vi "Dresden R2R Sputter 03.02.2018 IY24.vi"() -> ()   [LabVIEW 2009] (continued)
                n995 = local write "Casette_mechanism_1"(T/1 ("Casette_mechanism_4")) -> ()
                n996 = local write "Casette_mechanism_4"(i16? 0 ("Casette_mechanism_4")) -> ()
                n997 = local write "Casette_mechanism_3"(i16? 0 ("Casette_mechanism_3")) -> ()
                n998 = local write "Casette_mechanism_2"(i16? 0 ("Casette_mechanism_2")) -> ()
                "Ch1_tab_led" <- T/1 ("Ch1_tab_led")
                "Ch1_pump_tab_led" <- T/1 ("Ch1_pump_tab_led")
              }
              frame #2 {
                n999 = local write "ch_present_position"(dbl? 2.0 ("ch_present_position")) -> ()
                n1000 = local write "Casette_mechanism_2"(T/1 ("Casette_mechanism_2")) -> ()
                n1001 = local write "Casette_mechanism_1"(i16? 0 ("Casette_mechanism_4")) -> ()
                n1002 = local write "Casette_mechanism_4"(i16? 0 ("Casette_mechanism_4")) -> ()
                n1003 = local write "Casette_mechanism_3"(i16? 0 ("Casette_mechanism_3")) -> ()
                "Ch2_tab_led" <- T/1 ("Ch2_tab_led")
                "Ch2_pump_tab_led" <- T/1 ("Ch2_pump_tab_led")
              }
              frame #3 {
                n1004 = local write "ch_present_position"(dbl? 3.0 ("ch_present_position")) -> ()
                n1005 = local write "Casette_mechanism_3"(T/1 ("Casette_mechanism_3")) -> ()
                n1006 = local write "Casette_mechanism_2"(i16? 0 ("Casette_mechanism_2")) -> ()
                n1007 = local write "Casette_mechanism_1"(i16? 0 ("Casette_mechanism_4")) -> ()
                n1008 = local write "Casette_mechanism_4"(i16? 0 ("Casette_mechanism_4")) -> ()
                "Ch3_tab_led" <- T/1 ("Ch3_tab_led")
                "Ch3_pump_tab_led" <- T/1 ("Ch3_pump_tab_led")
              }
              frame #4 {
                n1009 = local write "ch_present_position"(dbl? 4.0 ("ch_present_position")) -> ()
                n1010 = local write "Casette_mechanism_4"(T/1 ("Casette_mechanism_4")) -> ()
                n1011 = local write "Casette_mechanism_3"(i16? 0 ("Casette_mechanism_3")) -> ()
                n1012 = local write "Casette_mechanism_2"(i16? 0 ("Casette_mechanism_2")) -> ()
                n1013 = local write "Casette_mechanism_1"(i16? 0 ("Casette_mechanism_4")) -> ()
                "Ch4_tab_led" <- T/1 ("Ch4_tab_led")
                "Ch4_pump_tab_led" <- T/1 ("Ch4_pump_tab_led")
              }
            }
            n1014 = Mantissa & Exponent(0:w1015) -> (2:w1013)  [unwired: 1 out]
            n1015 = case shown="1" w1013 {
              tunnel: [w1048 "Left" ("Casette_direction") "Right" ("Casette_direction")] -> w1012
              frame #0 {
                n1016 = local read "Casette_direction"() -> (w1048)
              }
              frame #1 {
              }
              frame #2 {
              }
            }
            "Casette_direction" <- w1012
          }
        }
      }
    }
  }
  n1017 = Build Path(base path="Gui_path", name or relative path="bv4 on.jpg") -> (appended path=w600:path)
  n1018 = Build Path(base path="Gui_path", name or relative path="bv4 fail.jpg") -> (appended path=w597:path)
  n1019 = Build Path(base path="Gui_path", name or relative path="gv on.jpg") -> (appended path=w605:path)
  n1020 = Build Path(base path="Gui_path", name or relative path="gv fail.jpg") -> (appended path=w608:path)
  n1021 = Build Path(base path="Gui_path", name or relative path="bv1 on.jpg") -> (appended path=w648:path)
  n1022 = Build Path(base path="Gui_path", name or relative path="vbv on.jpg") -> (appended path=w715:path)
  n1023 = Build Path(base path="Gui_path", name or relative path="bv1 fail.jpg") -> (appended path=w645:path)
  n1024 = Build Path(base path="Gui_path", name or relative path="mp on.jpg") -> (appended path=w728:path)
  n1025 = Build Path(base path="Gui_path", name or relative path="vbv fail.jpg") -> (appended path=w718:path)
  n1026 = Build Path(base path="Gui_path", name or relative path="mp fail.jpg") -> (appended path=w725:path)
  n1027 = Build Path(base path="Gui_path", name or relative path="pg on.jpg") -> (appended path=w712:path)
  n1028 = Build Path(base path="Gui_path", name or relative path="pg fail.jpg") -> (appended path=w709:path)
  n1029 = Build Path(base path="Gui_path", name or relative path="atm2 on.jpg") -> (appended path=w699:path)
  n1030 = Build Path(base path="Gui_path", name or relative path="atm2 fail.jpg") -> (appended path=w702:path)
  n1031 = Build Path(base path="Gui_path", name or relative path="bv1 on.jpg") -> (appended path=w696:path)
  n1032 = Build Path(base path="Gui_path", name or relative path="bv1 fail.jpg") -> (appended path=w693:path)
  n1033 = Build Path(base path="Gui_path", name or relative path="bv3 on.jpg") -> (appended path=w621:path)
  n1034 = Build Path(base path="Gui_path", name or relative path="vbv on.jpg") -> (appended path=w683:path)
  n1035 = Build Path(base path="Gui_path", name or relative path="bv3 fail.jpg") -> (appended path=w624:path)
  n1036 = Build Path(base path="Gui_path", name or relative path="vbv fail.jpg") -> (appended path=w686:path)
  n1037 = Build Path(base path="Gui_path", name or relative path="tp on.jpg") -> (appended path=w680:path)
  n1038 = Build Path(base path="Gui_path", name or relative path="tp fail.jpg") -> (appended path=w677:path)
  n1039 = Build Path(base path="Gui_path", name or relative path="tp gv on.jpg") -> (appended path=w667:path)
  n1040 = Build Path(base path="Gui_path", name or relative path="pg2 on.jpg") -> (appended path=w664:path)
  n1041 = Build Path(base path="Gui_path", name or relative path="tp gv fail.jpg") -> (appended path=w670:path)
  n1042 = Build Path(base path="Gui_path", name or relative path="tp gv middle.jpg") -> (appended path=w49:path)
  n1043 = Build Path(base path="Gui_path", name or relative path="pg2 fail.jpg") -> (appended path=w661:path)
  n1044 = Build Path(base path="Gui_path", name or relative path="bv2 on.jpg") -> (appended path=w618:path)
  n1045 = Build Path(base path="Gui_path", name or relative path="bv2 fail.jpg") -> (appended path=w615:path)
  n1046 = Build Path(base path="Gui_path", name or relative path="brt on.jpg") -> (appended path=w635:path)
  n1047 = Build Path(base path="Gui_path", name or relative path="brt fail.jpg") -> (appended path=w638:path)
  n1048 = Build Path(base path="Gui_path", name or relative path="atm3 on.jpg") -> (appended path=w632:path)
  n1049 = Build Path(base path="Gui_path", name or relative path="atm3 fail.jpg") -> (appended path=w629:path)
  n1050 = Build Path(base path="Gui_path", name or relative path="cc on.jpg") -> (appended path=w651:path)
  n1051 = Build Path(base path="Gui_path", name or relative path="cc fail.jpg") -> (appended path=w654:path)
  n1052 = Build Path(base path="Gui_path", name or relative path="bv5 on.jpg") -> (appended path=w591:path)
  n1053 = Build Path(base path="Gui_path", name or relative path="bv5 fail.jpg") -> (appended path=w594:path)
  n1054 = Build Path(base path="Gui_path", name or relative path="casette mechanism.jpg") -> (appended path=w42:path)
  n1055 = call <vilib>:"Read JPEG File.vi"("path to JPEG file"=w600) -> ("image data"=w601:T34)  [unwired: 8 in, 2 out]
  n1056 = call <vilib>:"Read JPEG File.vi"("path to JPEG file"=w597) -> ("image data"=w596:T34)  [unwired: 8 in, 2 out]
  n1057 = call <vilib>:"Read JPEG File.vi"("path to JPEG file"="Background_path") -> ("image data"=w732:T34)  [unwired: 8 in, 2 out]
  n1058 = call <vilib>:"Read JPEG File.vi"("path to JPEG file"=w605) -> ("image data"=w604:T34)  [unwired: 8 in, 2 out]
  n1059 = call <vilib>:"Read JPEG File.vi"("path to JPEG file"=w608) -> ("image data"=w609:T34)  [unwired: 8 in, 2 out]
  n1060 = call <vilib>:"Read JPEG File.vi"("path to JPEG file"=w648) -> ("image data"=w649:T34)  [unwired: 8 in, 2 out]
  n1061 = call <vilib>:"Read JPEG File.vi"("path to JPEG file"=w715) -> ("image data"=w714:T34)  [unwired: 8 in, 2 out]
  n1062 = call <vilib>:"Read JPEG File.vi"("path to JPEG file"=w645) -> ("image data"=w644:T34)  [unwired: 8 in, 2 out]
  n1063 = call <vilib>:"Read JPEG File.vi"("path to JPEG file"=w728) -> ("image data"=w729:T34)  [unwired: 8 in, 2 out]
  n1064 = call <vilib>:"Read JPEG File.vi"("path to JPEG file"=w718) -> ("image data"=w719:T34)  [unwired: 8 in, 2 out]
  n1065 = call <vilib>:"Read JPEG File.vi"("path to JPEG file"=w725) -> ("image data"=w724:T34)  [unwired: 8 in, 2 out]
  n1066 = call <vilib>:"Read JPEG File.vi"("path to JPEG file"=w712) -> ("image data"=w713:T34)  [unwired: 8 in, 2 out]
  n1067 = call <vilib>:"Read JPEG File.vi"("path to JPEG file"=w709) -> ("image data"=w708:T34)  [unwired: 8 in, 2 out]
  n1068 = call <vilib>:"Read JPEG File.vi"("path to JPEG file"=w699) -> ("image data"=w698:T34)  [unwired: 8 in, 2 out]
  n1069 = call <vilib>:"Read JPEG File.vi"("path to JPEG file"=w702) -> ("image data"=w703:T34)  [unwired: 8 in, 2 out]
  n1070 = call <vilib>:"Read JPEG File.vi"("path to JPEG file"=w696) -> ("image data"=w697:T34)  [unwired: 8 in, 2 out]
  n1071 = call <vilib>:"Read JPEG File.vi"("path to JPEG file"=w693) -> ("image data"=w692:T34)  [unwired: 8 in, 2 out]
  n1072 = call <vilib>:"Read JPEG File.vi"("path to JPEG file"=w621) -> ("image data"=w620:T34)  [unwired: 8 in, 2 out]
  n1073 = call <vilib>:"Read JPEG File.vi"("path to JPEG file"=w683) -> ("image data"=w682:T34)  [unwired: 8 in, 2 out]
  n1074 = call <vilib>:"Read JPEG File.vi"("path to JPEG file"=w624) -> ("image data"=w625:T34)  [unwired: 8 in, 2 out]
  n1075 = call <vilib>:"Read JPEG File.vi"("path to JPEG file"=w686) -> ("image data"=w687:T34)  [unwired: 8 in, 2 out]
  n1076 = call <vilib>:"Read JPEG File.vi"("path to JPEG file"=w680) -> ("image data"=w681:T34)  [unwired: 8 in, 2 out]
  n1077 = call <vilib>:"Read JPEG File.vi"("path to JPEG file"=w677) -> ("image data"=w676:T34)  [unwired: 8 in, 2 out]
  n1078 = call <vilib>:"Read JPEG File.vi"("path to JPEG file"=w667) -> ("image data"=w666:T34)  [unwired: 8 in, 2 out]
  n1079 = call <vilib>:"Read JPEG File.vi"("path to JPEG file"=w664) -> ("image data"=w665:T34)  [unwired: 8 in, 2 out]
  n1080 = call <vilib>:"Read JPEG File.vi"("path to JPEG file"=w670) -> ("image data"=w671:T34)  [unwired: 8 in, 2 out]
  n1081 = call <vilib>:"Read JPEG File.vi"("path to JPEG file"=w49) -> ("image data"=w48:T34)  [unwired: 8 in, 2 out]
  n1082 = call <vilib>:"Read JPEG File.vi"("path to JPEG file"=w661) -> ("image data"=w660:T34)  [unwired: 8 in, 2 out]
  n1083 = call <vilib>:"Read JPEG File.vi"("path to JPEG file"=w618) -> ("image data"=w619:T34)  [unwired: 8 in, 2 out]
  n1084 = call <vilib>:"Read JPEG File.vi"("path to JPEG file"=w615) -> ("image data"=w614:T34)  [unwired: 8 in, 2 out]
  n1085 = call <vilib>:"Read JPEG File.vi"("path to JPEG file"=w635) -> ("image data"=w634:T34)  [unwired: 8 in, 2 out]
  n1086 = call <vilib>:"Read JPEG File.vi"("path to JPEG file"=w638) -> ("image data"=w639:T34)  [unwired: 8 in, 2 out]
  n1087 = call <vilib>:"Read JPEG File.vi"("path to JPEG file"=w632) -> ("image data"=w633:T34)  [unwired: 8 in, 2 out]
  n1088 = call <vilib>:"Read JPEG File.vi"("path to JPEG file"=w629) -> ("image data"=w628:T34)  [unwired: 8 in, 2 out]
  n1089 = call <vilib>:"Read JPEG File.vi"("path to JPEG file"=w651) -> ("image data"=w650:T34)  [unwired: 8 in, 2 out]
  n1090 = call <vilib>:"Read JPEG File.vi"("path to JPEG file"=w654) -> ("image data"=w655:T34)  [unwired: 8 in, 2 out]
  n1091 = call <vilib>:"Read JPEG File.vi"("path to JPEG file"=w591) -> ("image data"=w590:T34)  [unwired: 8 in, 2 out]
  n1092 = call <vilib>:"Read JPEG File.vi"("path to JPEG file"=w594) -> ("image data"=w595:T34)  [unwired: 8 in, 2 out]
  n1093 = call <vilib>:"Read JPEG File.vi"("path to JPEG file"=w42) -> ("image data"=w45:T34)  [unwired: 8 in, 2 out]
  n1094 = call <vilib>:"Unflatten Pixmap.vi"("image data"=w601) -> ("24-bit pixmap"=w589:u32[][])  [unwired: 4 in, 6 out]
  n1095 = call <vilib>:"Unflatten Pixmap.vi"("image data"=w596) -> ("24-bit pixmap"=w588:u32[][])  [unwired: 4 in, 6 out]
  n1096 = call <vilib>:"Unflatten Pixmap.vi"("image data"=w732) -> ("24-bit pixmap"=w730:u32[][])  [unwired: 4 in, 6 out]
  n1097 = call <vilib>:"Unflatten Pixmap.vi"("image data"=w604) -> ("24-bit pixmap"=w603:u32[][])  [unwired: 4 in, 6 out]
  n1098 = call <vilib>:"Unflatten Pixmap.vi"("image data"=w609) -> ("24-bit pixmap"=w602:u32[][])  [unwired: 4 in, 6 out]
  n1099 = call <vilib>:"Unflatten Pixmap.vi"("image data"=w649) -> ("24-bit pixmap"=w643:u32[][])  [unwired: 4 in, 6 out]
  n1100 = call <vilib>:"Unflatten Pixmap.vi"("image data"=w714) -> ("24-bit pixmap"=w720:u32[][])  [unwired: 4 in, 6 out]
  n1101 = call <vilib>:"Unflatten Pixmap.vi"("image data"=w644) -> ("24-bit pixmap"=w642:u32[][])  [unwired: 4 in, 6 out]
  n1102 = call <vilib>:"Unflatten Pixmap.vi"("image data"=w729) -> ("24-bit pixmap"=w723:u32[][])  [unwired: 4 in, 6 out]
  n1103 = call <vilib>:"Unflatten Pixmap.vi"("image data"=w719) -> ("24-bit pixmap"=w721:u32[][])  [unwired: 4 in, 6 out]
  n1104 = call <vilib>:"Unflatten Pixmap.vi"("image data"=w724) -> ("24-bit pixmap"=w722:u32[][])  [unwired: 4 in, 6 out]
  n1105 = call <vilib>:"Unflatten Pixmap.vi"("image data"=w713) -> ("24-bit pixmap"=w707:u32[][])  [unwired: 4 in, 6 out]
  n1106 = call <vilib>:"Unflatten Pixmap.vi"("image data"=w708) -> ("24-bit pixmap"=w706:u32[][])  [unwired: 4 in, 6 out]
  n1107 = call <vilib>:"Unflatten Pixmap.vi"("image data"=w698) -> ("24-bit pixmap"=w704:u32[][])  [unwired: 4 in, 6 out]
  n1108 = call <vilib>:"Unflatten Pixmap.vi"("image data"=w703) -> ("24-bit pixmap"=w705:u32[][])  [unwired: 4 in, 6 out]
  n1109 = call <vilib>:"Unflatten Pixmap.vi"("image data"=w697) -> ("24-bit pixmap"=w691:u32[][])  [unwired: 4 in, 6 out]
  n1110 = call <vilib>:"Unflatten Pixmap.vi"("image data"=w692) -> ("24-bit pixmap"=w690:u32[][])  [unwired: 4 in, 6 out]
  n1111 = call <vilib>:"Unflatten Pixmap.vi"("image data"=w682) -> ("24-bit pixmap"=w688:u32[][])  [unwired: 4 in, 6 out]
  n1112 = call <vilib>:"Unflatten Pixmap.vi"("image data"=w687) -> ("24-bit pixmap"=w689:u32[][])  [unwired: 4 in, 6 out]
  n1113 = call <vilib>:"Unflatten Pixmap.vi"("image data"=w681) -> ("24-bit pixmap"=w675:u32[][])  [unwired: 4 in, 6 out]
  n1114 = call <vilib>:"Unflatten Pixmap.vi"("image data"=w620) -> ("24-bit pixmap"=w613:u32[][])  [unwired: 4 in, 6 out]
  n1115 = call <vilib>:"Unflatten Pixmap.vi"("image data"=w625) -> ("24-bit pixmap"=w612:u32[][])  [unwired: 4 in, 6 out]
  n1116 = call <vilib>:"Unflatten Pixmap.vi"("image data"=w676) -> ("24-bit pixmap"=w674:u32[][])  [unwired: 4 in, 6 out]
  n1117 = call <vilib>:"Unflatten Pixmap.vi"("image data"=w666) -> ("24-bit pixmap"=w672:u32[][])  [unwired: 4 in, 6 out]
  n1118 = call <vilib>:"Unflatten Pixmap.vi"("image data"=w665) -> ("24-bit pixmap"=w659:u32[][])  [unwired: 4 in, 6 out]
  n1119 = call <vilib>:"Unflatten Pixmap.vi"("image data"=w671) -> ("24-bit pixmap"=w673:u32[][])  [unwired: 4 in, 6 out]
  n1120 = call <vilib>:"Unflatten Pixmap.vi"("image data"=w48) -> ("24-bit pixmap"=w47:u32[][])  [unwired: 4 in, 6 out]
  n1121 = call <vilib>:"Unflatten Pixmap.vi"("image data"=w660) -> ("24-bit pixmap"=w658:u32[][])  [unwired: 4 in, 6 out]
  n1122 = call <vilib>:"Unflatten Pixmap.vi"("image data"=w634) -> ("24-bit pixmap"=w640:u32[][])  [unwired: 4 in, 6 out]
  n1123 = call <vilib>:"Unflatten Pixmap.vi"("image data"=w639) -> ("24-bit pixmap"=w641:u32[][])  [unwired: 4 in, 6 out]
  n1124 = call <vilib>:"Unflatten Pixmap.vi"("image data"=w619) -> ("24-bit pixmap"=w611:u32[][])  [unwired: 4 in, 6 out]
  n1125 = call <vilib>:"Unflatten Pixmap.vi"("image data"=w614) -> ("24-bit pixmap"=w610:u32[][])  [unwired: 4 in, 6 out]
  n1126 = call <vilib>:"Unflatten Pixmap.vi"("image data"=w633) -> ("24-bit pixmap"=w627:u32[][])  [unwired: 4 in, 6 out]
  n1127 = call <vilib>:"Unflatten Pixmap.vi"("image data"=w628) -> ("24-bit pixmap"=w626:u32[][])  [unwired: 4 in, 6 out]
  n1128 = call <vilib>:"Unflatten Pixmap.vi"("image data"=w650) -> ("24-bit pixmap"=w656:u32[][])  [unwired: 4 in, 6 out]
  n1129 = call <vilib>:"Unflatten Pixmap.vi"("image data"=w655) -> ("24-bit pixmap"=w657:u32[][])  [unwired: 4 in, 6 out]
  n1130 = call <vilib>:"Unflatten Pixmap.vi"("image data"=w590) -> ("24-bit pixmap"=w587:u32[][])  [unwired: 4 in, 6 out]
  n1131 = call <vilib>:"Unflatten Pixmap.vi"("image data"=w595) -> ("24-bit pixmap"=w586:u32[][])  [unwired: 4 in, 6 out]
  n1132 = call <vilib>:"Unflatten Pixmap.vi"("image data"=w45) -> ("24-bit pixmap"=w43:u32[][])  [unwired: 4 in, 6 out]
  n1133 = while {
    tunnel: w730 -> [w1872]
    tunnel: w723 -> [w1871]
    tunnel: w722 -> [w1870]
    tunnel: w720 -> [w1868]
    tunnel: w721 -> [w1869]
    tunnel: w707 -> [w1867]
    tunnel: w706 -> [w1866]
    tunnel: w704 -> [w1864]
    tunnel: w705 -> [w1865]
    tunnel: w691 -> [w1863]
    tunnel: w690 -> [w1862]
    tunnel: w688 -> [w1860]
    tunnel: w689 -> [w1861]
    tunnel: w675 -> [w1859]
    tunnel: w674 -> [w1858]
    tunnel: w672 -> [w1856]
    tunnel: w673 -> [w1857]
    tunnel: w659 -> [w1855]
    tunnel: w658 -> [w1854]
    tunnel: w656 -> [w1852]
    tunnel: w657 -> [w1853]
    tunnel: w643 -> [w1851]
    tunnel: w642 -> [w1850]
    tunnel: w640 -> [w1848]
    tunnel: w641 -> [w1849]
    tunnel: w627 -> [w1847]
    tunnel: w626 -> [w1846]
    tunnel: w613 -> [w1845]
    tunnel: w612 -> [w1844]
    tunnel: w611 -> [w1843]
    tunnel: w610 -> [w1842]
    tunnel: w603 -> [w1841]
    tunnel: w602 -> [w1840]
    tunnel: w589 -> [w1839]
    tunnel: w588 -> [w1838]
    tunnel: w587 -> [w1837]
    tunnel: w586 -> [w1836]
    tunnel: w47 -> [w1834]
    tunnel: w43 -> [w1833]
    stop <- FALSE stop-if-true
    n1134 = stacked-sequence {
      tunnel: w1872 -> [w1941 _ _]
      tunnel: w1871 -> [w2489 _ _]
      tunnel: w1870 -> [w2488 _ _]
      tunnel: w1868 -> [w2487 _ _]
      tunnel: w1869 -> [w2486 _ _]
      tunnel: w1867 -> [w2484 _ _]
      tunnel: w1866 -> [w2485 _ _]
      tunnel: w1864 -> [w2420 _ _]
      tunnel: w1865 -> [w2419 _ _]
      tunnel: w1863 -> [w2416 _ _]
      tunnel: w1862 -> [w2417 _ _]
      tunnel: w1860 -> [w2352 _ _]
      tunnel: w1861 -> [w2351 _ _]
      tunnel: w1859 -> [w2348 _ _]
      tunnel: w1858 -> [w2349 _ _]
      tunnel: w1856 -> [w2284 _ _]
      tunnel: w1857 -> [w2283 _ _]
      tunnel: w1855 -> [w2280 _ _]
      tunnel: w1854 -> [w2281 _ _]
      tunnel: w1852 -> [w2216 _ _]
      tunnel: w1853 -> [w2215 _ _]
      tunnel: w1851 -> [w2212 _ _]
      tunnel: w1850 -> [w2213 _ _]
      tunnel: w1848 -> [w2148 _ _]
      tunnel: w1849 -> [w2147 _ _]
      tunnel: w1847 -> [w2066 _ _]
      tunnel: w1846 -> [w2118 _ _]
      tunnel: w1845 -> [w2065 _ _]
      tunnel: w1844 -> [w2064 _ _]
      tunnel: w1843 -> [w2063 _ _]
      tunnel: w1842 -> [w2062 _ _]
      tunnel: w1841 -> [w2037 _ _]
      tunnel: w1840 -> [w2036 _ _]
      tunnel: w1839 -> [w1989 _ _]
      tunnel: w1838 -> [w1988 _ _]
      tunnel: w1837 -> [w1987 _ _]
      tunnel: w1836 -> [w1986 _ _]
      tunnel: [_ w3353 _] -> w1835
      tunnel: w1834 -> [w1979 _ _]
      tunnel: w1833 -> [w1947 _ _]
      frame #0 {
        n1135 = Build Array(FALSE ("element"), "Ch1_Mp_on", "Ch1_Mp_fail") -> (w2549:bool[])
        n1136 = Build Array(FALSE ("element"), "Ch2_Mp_on", "Ch2_Mp_fail") -> (w2541:bool[])
        n1137 = Build Array(FALSE ("element"), "Ch3_Mp_on", "Ch3_Mp_fail") -> (w2533:bool[])
        n1138 = Build Array(FALSE ("element"), "Ch4_Mp_on", "Ch4_Mp_fail") -> (w2525:bool[])
        n1139 = Build Array(FALSE ("element"), "Ch1_Pl_vbv_on", "Ch1_Pl_vbv_fail") -> (w2494:bool[])
        n1140 = Build Array(FALSE ("element"), "Ch2_Pl_vbv_on", "Ch2_Pl_vbv_fail") -> (w2501:bool[])
        n1141 = Build Array(FALSE ("element"), "Ch3_Pl_vbv_on", "Ch3_Pl_vbv_fail") -> (w2509:bool[])
        n1142 = Build Array(FALSE ("element"), "Ch4_Pl_vbv_on", "Ch4_Pl_vbv_fail") -> (w2517:bool[])
        n1143 = Build Array(FALSE ("element"), "Ch1_Pl_pg_on", "Ch1_Pl_pg_fail") -> (w2480:bool[])
        n1144 = Build Array(FALSE ("element"), "Ch2_Pl_pg_on", "Ch2_Pl_pg_fail") -> (w2473:bool[])
        n1145 = Build Array(FALSE ("element"), "Ch3_Pl_pg_on", "Ch3_Pl_pg_fail") -> (w2465:bool[])
        n1146 = Build Array(FALSE ("element"), "Ch4_Pl_pg_on", "Ch4_Pl_pg_fail") -> (w2457:bool[])
        n1147 = Build Array(FALSE ("element"), "Ch1_Pl_atm_on", "Ch1_Pl_atm_fail") -> (w2424:bool[])
        n1148 = Build Array(FALSE ("element"), "Ch2_Pl_atm_on", "Ch2_Pl_atm_fail") -> (w2431:bool[])
        n1149 = Build Array(FALSE ("element"), "Ch3_Pl_atm_on", "Ch3_Pl_atm_fail") -> (w2439:bool[])
        n1150 = Build Array(FALSE ("element"), "Ch4_Pl_atm_on", "Ch4_Pl_atm_fail") -> (w2447:bool[])
        n1151 = Build Array(FALSE ("element"), "Ch1_Tp_bv_on", "Ch1_Tp_bv_fail") -> (w2412:bool[])
        n1152 = Build Array(FALSE ("element"), "Ch2_Tp_bv_on", "Ch2_Tp_bv_fail") -> (w2405:bool[])
        n1153 = Build Array(FALSE ("element"), "Ch3_Tp_bv_on", "Ch3_Tp_bv_fail") -> (w2397:bool[])
        n1154 = Build Array(FALSE ("element"), "Ch4_Tp_bv_on", "Ch4_Tp_bv_fail") -> (w2389:bool[])
        n1155 = Build Array(FALSE ("element"), "Ch1_Ch_vbv_on", "Ch1_Ch_vbv_fail") -> (w2356:bool[])
        n1156 = Build Array(FALSE ("element"), "Ch2_Ch_vbv_on", "Ch2_Ch_vbv_fail") -> (w2363:bool[])
        n1157 = Build Array(FALSE ("element"), "Ch3_Ch_vbv_on", "Ch3_Ch_vbv_fail") -> (w2371:bool[])
        n1158 = Build Array(FALSE ("element"), "Ch4_Ch_vbv_on", "Ch4_Ch_vbv_fail") -> (w2379:bool[])
        n1159 = Build Array(FALSE ("element"), "Ch1_Tp_on", "Ch1_Tp_fail") -> (w2344:bool[])
        n1160 = Build Array(FALSE ("element"), "Ch2_Tp_on", "Ch2_Tp_fail") -> (w2337:bool[])
        n1161 = Build Array(FALSE ("element"), "Ch3_Tp_on", "Ch3_Tp_fail") -> (w2329:bool[])
        n1162 = Build Array(FALSE ("element"), "Ch4_Tp_on", "Ch4_Tp_fail") -> (w2321:bool[])
        n1163 = Build Array(FALSE ("element"), "Ch1_Pc_bv_on", "Ch1_Pc_bv_fail", "Ch1_Pc_bv_middle") -> (w2288:bool[])
        n1164 = Build Array(FALSE ("element"), "Ch2_Pc_bv_on", "Ch2_Pc_bv_fail", "Ch2_Pc_bv_middle") -> (w2295:bool[])
        n1165 = Build Array(FALSE ("element"), "Ch3_Pc_bv_on", "Ch3_Pc_bv_fail", "Ch3_Pc_bv_middle") -> (w2303:bool[])
        n1166 = Build Array(FALSE ("element"), "Ch4_Pc_bv_on", "Ch4_Pc_bv_fail", "Ch4_Pc_bv_middle") -> (w2311:bool[])
        n1167 = Build Array(FALSE ("element"), "Ch1_Ch_pg_on", "Ch1_Ch_pg_fail") -> (w2276:bool[])
        n1168 = Build Array(FALSE ("element"), "Ch2_Ch_pg_on", "Ch2_Ch_pg_fail") -> (w2269:bool[])
        n1169 = Build Array(FALSE ("element"), "Ch3_Ch_pg_on", "Ch3_Ch_pg_fail") -> (w2261:bool[])
        n1170 = Build Array(FALSE ("element"), "Ch4_Ch_pg_on", "Ch4_Ch_pg_fail") -> (w2253:bool[])
        n1171 = Build Array(FALSE ("element"), "Ch1_Ch_cc_on", "Ch1_Ch_cc_fail") -> (w2220:bool[])
        n1172 = Build Array(FALSE ("element"), "Ch2_Ch_cc_on", "Ch2_Ch_cc_fail") -> (w2227:bool[])
        n1173 = Build Array(FALSE ("element"), "Ch3_Ch_cc_on", "Ch3_Ch_cc_fail") -> (w2235:bool[])
        n1174 = Build Array(FALSE ("element"), "Ch4_Ch_cc_on", "Ch4_Ch_cc_fail") -> (w2243:bool[])
        n1175 = Build Array(FALSE ("element"), "Ch1_Bg_bv_on", "Ch1_Bg_bv_fail") -> (w2208:bool[])
        n1176 = Build Array(FALSE ("element"), "Ch2_Bg_bv_on", "Ch2_Bg_bv_fail") -> (w2201:bool[])
        n1177 = Build Array(FALSE ("element"), "Ch3_Bg_bv_on", "Ch3_Bg_bv_fail") -> (w2193:bool[])
        n1178 = Build Array(FALSE ("element"), "Ch1_Ch_bg_on", "Ch1_Ch_bg_fail") -> (w2152:bool[])
        n1179 = Build Array(FALSE ("element"), "Ch4_Bg_bv_on", "Ch4_Bg_bv_fail") -> (w2185:bool[])
        n1180 = Build Array(FALSE ("element"), "Ch2_Ch_bg_on", "Ch2_Ch_bg_fail") -> (w2159:bool[])
        n1181 = Build Array(FALSE ("element"), "Ch3_Ch_bg_on", "Ch3_Ch_bg_fail") -> (w2167:bool[])
        n1182 = Build Array(FALSE ("element"), "Ch1_Ch_atm_on", "Ch1_Ch_atm_fail") -> (w2142:bool[])
        n1183 = Build Array(FALSE ("element"), "Ch4_Ch_bg_on", "Ch4_Ch_bg_fail") -> (w2175:bool[])
        n1184 = Build Array(FALSE ("element"), "Ch2_Ch_atm_on", "Ch2_Ch_atm_fail") -> (w2137:bool[])
        n1185 = Build Array(FALSE ("element"), "Ch3_Ch_atm_on", "Ch3_Ch_atm_fail") -> (w2134:bool[])
        n1186 = Build Array(FALSE ("element"), "Ch4_Ch_atm_on", "Ch4_Ch_atm_fail") -> (w2133:bool[])
        n1187 = Build Array(FALSE ("element"), "Ch1_Trns_gv_bp2_on", "Ch1_Trns_gv_bp2_fail") -> (w2111:bool[])
        n1188 = Build Array(FALSE ("element"), "Ch2_Trns_gv_bp2_on", "Ch2_Trns_gv_bp2_fail") -> (w2110:bool[])
        n1189 = Build Array(FALSE ("element"), "Ch3_Trns_gv_bp2_on", "Ch3_Trns_gv_bp2_fail") -> (w2103:bool[])
        n1190 = Build Array(FALSE ("element"), "Ch2_Trns_gv_bp_on", "Ch2_Trns_gv_bp_fail") -> (w2102:bool[])
        n1191 = Build Array(FALSE ("element"), "Ch4_Trns_gv_bp_on", "Ch4_Trns_gv_bp_fail") -> (w2094:bool[])
        n1192 = Build Array(FALSE ("element"), "Ch3_Trns_gv_bp_on", "Ch3_Trns_gv_bp_fail") -> (w2095:bool[])
        n1193 = Build Array(FALSE ("element"), "Trns_gv_1_2_on", "Trns_gv1_2_fail") -> (w2058:bool[])
        n1194 = Build Array(FALSE ("element"), "Trns_gv_2_3_on", "Trns_gv_2_3_fail") -> (w2057:bool[])
        n1195 = Build Array(FALSE ("element"), "Trns_gv_3_4_on", "Trns_gv_3_4_fail") -> (w2050:bool[])
        n1196 = Build Array(FALSE ("element"), "Ch1_Bp_bv_fail_R", "Ch1_Bp_bv_on_R") -> (w2035:bool[])
        n1197 = Build Array(FALSE ("element"), "Ch2_Bp_bv_on_R", "Ch2_Bp_bv_fail_R") -> (w2028:bool[])
        n1198 = Build Array(FALSE ("element"), "Ch3_Bp_bv_on_R", "Ch3_Bp_bv_fail_R") -> (w2027:bool[])
        n1199 = Build Array(FALSE ("element"), "Ch2_Bp_bv_on_L", "Ch2_Bp_bv_fail_L") -> (w2020:bool[])
        n1200 = Build Array(FALSE ("element"), "Ch3_Bp_bv_on_L", "Ch3_Bp_bv_fail_L") -> (w2019:bool[])
        n1201 = Build Array(FALSE ("element"), "Ch4_Bp_bv_on_L", "Ch4_Bp_bv_fail_L") -> (w2012:bool[])
        n1202 = Boolean Array To Number(Boolean array=w2549) -> (number=w2548:u32)
        n1203 = Boolean Array To Number(Boolean array=w2541) -> (number=w2542:u32)
        n1204 = Boolean Array To Number(Boolean array=w2533) -> (number=w2532:u32)
        n1205 = Build Array(FALSE ("element"), "Casette_mechanism_4") -> (w1978:bool[])
        n1206 = Boolean Array To Number(Boolean array=w2525) -> (number=w2526:u32)
        n1207 = Boolean Array To Number(Boolean array=w2494) -> (number=w2495:u32)
        n1208 = Build Array(FALSE ("element"), "Casette_mechanism_3") -> (w1964:bool[])
        n1209 = Build Array(FALSE ("element"), "Casette_mechanism_2") -> (w1962:bool[])
        n1210 = Boolean Array To Number(Boolean array=w2501) -> (number=w2500:u32)
        n1211 = Boolean Array To Number(Boolean array=w2509) -> (number=w2510:u32)
        n1212 = Build Array(FALSE ("element"), "Casette_mechanism_1") -> (w1948:bool[])
        n1213 = Boolean Array To Number(Boolean array=w2517) -> (number=w2516:u32)
        n1214 = Boolean Array To Number(Boolean array=w2480) -> (number=w2479:u32)
        n1215 = Boolean Array To Number(Boolean array=w2473) -> (number=w2474:u32)
        n1216 = Boolean Array To Number(Boolean array=w2465) -> (number=w2464:u32)
        n1217 = Boolean Array To Number(Boolean array=w2457) -> (number=w2458:u32)
        n1218 = Boolean Array To Number(Boolean array=w2424) -> (number=w2425:u32)
        n1219 = Boolean Array To Number(Boolean array=w2431) -> (number=w2430:u32)
        n1220 = Boolean Array To Number(Boolean array=w2439) -> (number=w2440:u32)
        n1221 = Boolean Array To Number(Boolean array=w2447) -> (number=w2446:u32)
        n1222 = Boolean Array To Number(Boolean array=w2412) -> (number=w2411:u32)
        n1223 = Boolean Array To Number(Boolean array=w2405) -> (number=w2406:u32)
        n1224 = Boolean Array To Number(Boolean array=w2397) -> (number=w2396:u32)
        n1225 = Boolean Array To Number(Boolean array=w2389) -> (number=w2390:u32)
        n1226 = Boolean Array To Number(Boolean array=w2356) -> (number=w2357:u32)
        n1227 = Boolean Array To Number(Boolean array=w2363) -> (number=w2362:u32)
        n1228 = Boolean Array To Number(Boolean array=w2371) -> (number=w2372:u32)
        n1229 = Boolean Array To Number(Boolean array=w2379) -> (number=w2378:u32)
        n1230 = Boolean Array To Number(Boolean array=w2344) -> (number=w2343:u32)
        n1231 = Boolean Array To Number(Boolean array=w2337) -> (number=w2338:u32)
        n1232 = Boolean Array To Number(Boolean array=w2329) -> (number=w2328:u32)
        n1233 = Boolean Array To Number(Boolean array=w2321) -> (number=w2322:u32)
        n1234 = Boolean Array To Number(Boolean array=w2288) -> (number=w2289:u32)
        n1235 = Boolean Array To Number(Boolean array=w2295) -> (number=w2294:u32)
        n1236 = Boolean Array To Number(Boolean array=w2303) -> (number=w2304:u32)
        n1237 = Boolean Array To Number(Boolean array=w2311) -> (number=w2310:u32)
        n1238 = Boolean Array To Number(Boolean array=w2276) -> (number=w2275:u32)
        n1239 = Boolean Array To Number(Boolean array=w2269) -> (number=w2270:u32)
        n1240 = Boolean Array To Number(Boolean array=w2261) -> (number=w2260:u32)
        n1241 = Boolean Array To Number(Boolean array=w2253) -> (number=w2254:u32)
        n1242 = Boolean Array To Number(Boolean array=w2220) -> (number=w2221:u32)
        n1243 = Boolean Array To Number(Boolean array=w2227) -> (number=w2226:u32)
        n1244 = Boolean Array To Number(Boolean array=w2235) -> (number=w2236:u32)
        n1245 = Boolean Array To Number(Boolean array=w2243) -> (number=w2242:u32)
        n1246 = Boolean Array To Number(Boolean array=w2208) -> (number=w2207:u32)
        n1247 = Boolean Array To Number(Boolean array=w2201) -> (number=w2202:u32)
        n1248 = Boolean Array To Number(Boolean array=w2193) -> (number=w2192:u32)
        n1249 = Boolean Array To Number(Boolean array=w2152) -> (number=w2153:u32)
        n1250 = Boolean Array To Number(Boolean array=w2185) -> (number=w2186:u32)
        n1251 = Boolean Array To Number(Boolean array=w2159) -> (number=w2158:u32)
        n1252 = Boolean Array To Number(Boolean array=w2167) -> (number=w2168:u32)
        n1253 = Boolean Array To Number(Boolean array=w2142) -> (number=w2143:u32)
        n1254 = Boolean Array To Number(Boolean array=w2175) -> (number=w2174:u32)
        n1255 = Boolean Array To Number(Boolean array=w2137) -> (number=w2136:u32)
        n1256 = Boolean Array To Number(Boolean array=w2134) -> (number=w2135:u32)
        n1257 = Boolean Array To Number(Boolean array=w2133) -> (number=w2132:u32)
        n1258 = Boolean Array To Number(Boolean array=w2111) -> (number=w2112:u32)
        n1259 = Boolean Array To Number(Boolean array=w2110) -> (number=w2109:u32)
        n1260 = Boolean Array To Number(Boolean array=w2103) -> (number=w2104:u32)
        n1261 = Boolean Array To Number(Boolean array=w2102) -> (number=w2101:u32)
        n1262 = Boolean Array To Number(Boolean array=w2094) -> (number=w2093:u32)
        n1263 = Boolean Array To Number(Boolean array=w2095) -> (number=w2096:u32)
        n1264 = Boolean Array To Number(Boolean array=w2058) -> (number=w2059:u32)
        n1265 = Boolean Array To Number(Boolean array=w2057) -> (number=w2056:u32)
        n1266 = Boolean Array To Number(Boolean array=w2050) -> (number=w2051:u32)
        n1267 = Boolean Array To Number(Boolean array=w2035) -> (number=w2034:u32)
        n1268 = Boolean Array To Number(Boolean array=w2028) -> (number=w2029:u32)
        n1269 = Boolean Array To Number(Boolean array=w2027) -> (number=w2026:u32)
        n1270 = Boolean Array To Number(Boolean array=w2020) -> (number=w2021:u32)
        n1271 = Boolean Array To Number(Boolean array=w2019) -> (number=w2018:u32)
        n1272 = Boolean Array To Number(Boolean array=w2012) -> (number=w2013:u32)
        n1273 = Boolean Array To Number(Boolean array=w1978) -> (number=w1977:u32)
        n1274 = Boolean Array To Number(Boolean array=w1964) -> (number=w1965:u32)
        n1275 = Boolean Array To Number(Boolean array=w1962) -> (number=w1961:u32)
        n1276 = Boolean Array To Number(Boolean array=w1948) -> (number=w1949:u32)
        n1277 = Mantissa & Exponent(0:w2548) -> (2:w2547:dbl)  [unwired: 1 out]
        n1278 = Mantissa & Exponent(0:w2542) -> (2:w2543:dbl)  [unwired: 1 out]
        n1279 = Mantissa & Exponent(0:w2532) -> (2:w2531:dbl)  [unwired: 1 out]
        n1280 = Mantissa & Exponent(0:w2526) -> (2:w2527:dbl)  [unwired: 1 out]
        n1281 = Mantissa & Exponent(0:w2495) -> (2:w2496:dbl)  [unwired: 1 out]
        n1282 = Mantissa & Exponent(0:w2500) -> (2:w2499:dbl)  [unwired: 1 out]
        n1283 = Mantissa & Exponent(0:w2510) -> (2:w2511:dbl)  [unwired: 1 out]
        n1284 = Mantissa & Exponent(0:w2516) -> (2:w2515:dbl)  [unwired: 1 out]
        n1285 = Mantissa & Exponent(0:w2479) -> (2:w2478:dbl)  [unwired: 1 out]
        n1286 = Mantissa & Exponent(0:w2474) -> (2:w2475:dbl)  [unwired: 1 out]
        n1287 = Mantissa & Exponent(0:w2464) -> (2:w2463:dbl)  [unwired: 1 out]
        n1288 = Mantissa & Exponent(0:w2458) -> (2:w2459:dbl)  [unwired: 1 out]
        n1289 = Mantissa & Exponent(0:w2425) -> (2:w2426:dbl)  [unwired: 1 out]
        n1290 = Mantissa & Exponent(0:w2430) -> (2:w2429:dbl)  [unwired: 1 out]
        n1291 = Mantissa & Exponent(0:w2440) -> (2:w2441:dbl)  [unwired: 1 out]
        n1292 = Mantissa & Exponent(0:w2446) -> (2:w2445:dbl)  [unwired: 1 out]
        n1293 = Mantissa & Exponent(0:w2411) -> (2:w2410:dbl)  [unwired: 1 out]
        n1294 = Mantissa & Exponent(0:w2406) -> (2:w2407:dbl)  [unwired: 1 out]
        n1295 = Mantissa & Exponent(0:w2396) -> (2:w2395:dbl)  [unwired: 1 out]
        n1296 = Mantissa & Exponent(0:w2390) -> (2:w2391:dbl)  [unwired: 1 out]
        n1297 = Mantissa & Exponent(0:w2357) -> (2:w2358:dbl)  [unwired: 1 out]
        n1298 = Mantissa & Exponent(0:w2362) -> (2:w2361:dbl)  [unwired: 1 out]
        n1299 = Mantissa & Exponent(0:w2372) -> (2:w2373:dbl)  [unwired: 1 out]
        n1300 = Mantissa & Exponent(0:w2378) -> (2:w2377:dbl)  [unwired: 1 out]
        n1301 = Mantissa & Exponent(0:w2343) -> (2:w2342:dbl)  [unwired: 1 out]
        n1302 = Mantissa & Exponent(0:w2338) -> (2:w2339:dbl)  [unwired: 1 out]
        n1303 = Mantissa & Exponent(0:w2328) -> (2:w2327:dbl)  [unwired: 1 out]
        n1304 = Mantissa & Exponent(0:w2322) -> (2:w2323:dbl)  [unwired: 1 out]
        n1305 = Mantissa & Exponent(0:w2289) -> (2:w2290:dbl)  [unwired: 1 out]
        n1306 = Mantissa & Exponent(0:w2294) -> (2:w2293:dbl)  [unwired: 1 out]
        n1307 = Mantissa & Exponent(0:w2304) -> (2:w2305:dbl)  [unwired: 1 out]
        n1308 = Mantissa & Exponent(0:w2310) -> (2:w2309:dbl)  [unwired: 1 out]
        n1309 = Mantissa & Exponent(0:w2275) -> (2:w2274:dbl)  [unwired: 1 out]
        n1310 = Mantissa & Exponent(0:w2270) -> (2:w2271:dbl)  [unwired: 1 out]
        n1311 = Mantissa & Exponent(0:w2260) -> (2:w2259:dbl)  [unwired: 1 out]
        n1312 = Mantissa & Exponent(0:w2254) -> (2:w2255:dbl)  [unwired: 1 out]
        n1313 = Mantissa & Exponent(0:w2221) -> (2:w2222:dbl)  [unwired: 1 out]
        n1314 = Mantissa & Exponent(0:w2226) -> (2:w2225:dbl)  [unwired: 1 out]
        n1315 = Mantissa & Exponent(0:w2236) -> (2:w2237:dbl)  [unwired: 1 out]
        n1316 = Mantissa & Exponent(0:w2242) -> (2:w2241:dbl)  [unwired: 1 out]
        n1317 = Mantissa & Exponent(0:w2207) -> (2:w2206:dbl)  [unwired: 1 out]
        n1318 = Mantissa & Exponent(0:w2202) -> (2:w2203:dbl)  [unwired: 1 out]
        n1319 = Mantissa & Exponent(0:w2192) -> (2:w2191:dbl)  [unwired: 1 out]
        n1320 = Mantissa & Exponent(0:w2153) -> (2:w2154:dbl)  [unwired: 1 out]
        n1321 = Mantissa & Exponent(0:w2186) -> (2:w2187:dbl)  [unwired: 1 out]
        n1322 = Mantissa & Exponent(0:w2158) -> (2:w2157:dbl)  [unwired: 1 out]
        n1323 = Mantissa & Exponent(0:w2168) -> (2:w2169:dbl)  [unwired: 1 out]
        n1324 = Mantissa & Exponent(0:w2143) -> (2:w2141:dbl)  [unwired: 1 out]
        n1325 = Mantissa & Exponent(0:w2174) -> (2:w2173:dbl)  [unwired: 1 out]
        n1326 = Mantissa & Exponent(0:w2136) -> (2:w2131:dbl)  [unwired: 1 out]
        n1327 = Mantissa & Exponent(0:w2135) -> (2:w2130:dbl)  [unwired: 1 out]
        n1328 = Mantissa & Exponent(0:w2132) -> (2:w2129:dbl)  [unwired: 1 out]
        n1329 = Mantissa & Exponent(0:w2112) -> (2:w2113:dbl)  [unwired: 1 out]
        n1330 = Mantissa & Exponent(0:w2109) -> (2:w2108:dbl)  [unwired: 1 out]
        n1331 = Mantissa & Exponent(0:w2104) -> (2:w2105:dbl)  [unwired: 1 out]
        n1332 = Mantissa & Exponent(0:w2101) -> (2:w2100:dbl)  [unwired: 1 out]
        n1333 = Mantissa & Exponent(0:w2093) -> (2:w2092:dbl)  [unwired: 1 out]
        n1334 = Mantissa & Exponent(0:w2096) -> (2:w2097:dbl)  [unwired: 1 out]
        n1335 = Mantissa & Exponent(0:w2059) -> (2:w2060:dbl)  [unwired: 1 out]
        n1336 = Mantissa & Exponent(0:w2056) -> (2:w2055:dbl)  [unwired: 1 out]
        n1337 = Mantissa & Exponent(0:w2051) -> (2:w2052:dbl)  [unwired: 1 out]
        n1338 = Mantissa & Exponent(0:w2034) -> (2:w2033:dbl)  [unwired: 1 out]
        n1339 = Mantissa & Exponent(0:w2029) -> (2:w2030:dbl)  [unwired: 1 out]
        n1340 = Mantissa & Exponent(0:w2026) -> (2:w2025:dbl)  [unwired: 1 out]
        n1341 = Mantissa & Exponent(0:w2021) -> (2:w2022:dbl)  [unwired: 1 out]
        n1342 = Mantissa & Exponent(0:w2018) -> (2:w2017:dbl)  [unwired: 1 out]
        n1343 = Mantissa & Exponent(0:w2013) -> (2:w2014:dbl)  [unwired: 1 out]
        n1344 = Mantissa & Exponent(0:w1977) -> (2:w1974:dbl)  [unwired: 1 out]
        n1345 = Mantissa & Exponent(0:w1965) -> (2:w1968:dbl)  [unwired: 1 out]
        n1346 = Mantissa & Exponent(0:w1961) -> (2:w1958:dbl)  [unwired: 1 out]
        n1347 = Mantissa & Exponent(0:w1949) -> (2:w1952:dbl)  [unwired: 1 out]
        n1348 = case shown="1" w2547 {
          tunnel: w2489 -> [_ w2764 _]
          tunnel: w2488 -> [_ _ w2765]
          tunnel: [u32[][] [] ("24-bit pixmap") w2764 w2765] -> w2545
          frame #0 {
          }
          frame #1 {
          }
          frame #2 {
          }
        }
        n1349 = case shown="0, Default" w2543 {
          tunnel: w2489 -> [_ w2761 _]
          tunnel: w2488 -> [_ _ w2762]
          tunnel: [u32[][] [] ("24-bit pixmap") w2761 w2762] -> w2544
          frame #0 {
          }
          frame #1 {
          }
          frame #2 {
          }
        }
        n1350 = case shown="0, Default" w2531 {
          tunnel: w2489 -> [_ w2758 _]
          tunnel: w2488 -> [_ _ w2759]
          tunnel: [u32[][] [] ("24-bit pixmap") w2758 w2759] -> w2530
          frame #0 {
          }
          frame #1 {
          }
          frame #2 {
          }
        }
        n1351 = case shown="0, Default" w2527 {
          tunnel: w2489 -> [_ w2755 _]
          tunnel: w2488 -> [_ _ w2756]
          tunnel: [u32[][] [] ("24-bit pixmap") w2755 w2756] -> w2528
          frame #0 {
          }
          frame #1 {
          }
          frame #2 {
          }
        }
        n1352 = case shown="0, Default" w2496 {
          tunnel: w2487 -> [_ w2752 _]
          tunnel: w2486 -> [_ _ w2753]
          tunnel: [u32[][] [] ("24-bit pixmap") w2752 w2753] -> w2497
          frame #0 {
          }
          frame #1 {
          }
          frame #2 {
          }
        }
        n1353 = case shown="0, Default" w2499 {
          tunnel: w2487 -> [_ w2749 _]
          tunnel: w2486 -> [_ _ w2750]
          tunnel: [u32[][] [] ("24-bit pixmap") w2749 w2750] -> w2498
          frame #0 {
          }
          frame #1 {
          }
          frame #2 {
          }
        }
        n1354 = case shown="0, Default" w2511 {
          tunnel: w2487 -> [_ w2746 _]
          tunnel: w2486 -> [_ _ w2747]
          tunnel: [u32[][] [] ("24-bit pixmap") w2746 w2747] -> w2512
          frame #0 {
          }
          frame #1 {
          }
          frame #2 {
          }
        }
        n1355 = case shown="0, Default" w2515 {
          tunnel: w2487 -> [_ w2743 _]
          tunnel: w2486 -> [_ _ w2744]
          tunnel: [u32[][] [] ("24-bit pixmap") w2743 w2744] -> w2514
          frame #0 {
          }
          frame #1 {
          }
          frame #2 {
          }
        }
        n1356 = case shown="2" w2478 {
          tunnel: w2484 -> [_ w2740 _]
          tunnel: w2485 -> [_ _ w2741]
          tunnel: [u32[][] [] ("24-bit pixmap") w2740 w2741] -> w2477
          frame #0 {
          }
          frame #1 {
          }
          frame #2 {
          }
        }
        n1357 = case shown="0, Default" w2475 {
          tunnel: w2484 -> [_ w2737 _]
          tunnel: w2485 -> [_ _ w2738]
          tunnel: [u32[][] [] ("24-bit pixmap") w2737 w2738] -> w2476
          frame #0 {
          }
          frame #1 {
          }
          frame #2 {
          }
        }
        n1358 = case shown="0, Default" w2463 {
          tunnel: w2484 -> [_ w2734 _]
          tunnel: w2485 -> [_ _ w2735]
          tunnel: [u32[][] [] ("24-bit pixmap") w2734 w2735] -> w2462
          frame #0 {
          }
          frame #1 {
          }
          frame #2 {
          }
        }
        n1359 = case shown="0, Default" w2459 {
          tunnel: w2484 -> [_ w2731 _]
          tunnel: w2485 -> [_ _ w2732]
          tunnel: [u32[][] [] ("24-bit pixmap") w2731 w2732] -> w2460
          frame #0 {
          }
          frame #1 {
          }
          frame #2 {
          }
        }
        n1360 = case shown="0, Default" w2426 {
          tunnel: w2420 -> [_ w2728 _]
          tunnel: w2419 -> [_ _ w2729]
          tunnel: [u32[][] [] ("24-bit pixmap") w2728 w2729] -> w2427
          frame #0 {
          }
          frame #1 {
          }
          frame #2 {
          }
        }
        n1361 = case shown="0, Default" w2429 {
          tunnel: w2420 -> [_ w2725 _]
          tunnel: w2419 -> [_ _ w2726]
          tunnel: [u32[][] [] ("24-bit pixmap") w2725 w2726] -> w2428
          frame #0 {
          }
          frame #1 {
          }
          frame #2 {
          }
        }
        n1362 = case shown="0, Default" w2441 {
          tunnel: w2420 -> [_ w2722 _]
          tunnel: w2419 -> [_ _ w2723]
          tunnel: [u32[][] [] ("24-bit pixmap") w2722 w2723] -> w2442
          frame #0 {
          }
          frame #1 {
          }
          frame #2 {
          }
        }
        n1363 = case shown="0, Default" w2445 {
          tunnel: w2420 -> [_ w2719 _]
          tunnel: w2419 -> [_ _ w2720]
          tunnel: [u32[][] [] ("24-bit pixmap") w2719 w2720] -> w2444
          frame #0 {
          }
          frame #1 {
          }
          frame #2 {
          }
        }
        n1364 = case shown="0, Default" w2410 {
          tunnel: w2416 -> [_ w2716 _]
          tunnel: w2417 -> [_ _ w2717]
          tunnel: [u32[][] [] ("24-bit pixmap") w2716 w2717] -> w2409
          frame #0 {
          }
          frame #1 {
          }
          frame #2 {
          }
        }
        n1365 = case shown="0, Default" w2407 {
          tunnel: w2416 -> [_ w2713 _]
          tunnel: w2417 -> [_ _ w2714]
          tunnel: [u32[][] [] ("24-bit pixmap") w2713 w2714] -> w2408
          frame #0 {
          }
          frame #1 {
          }
          frame #2 {
          }
        }
        n1366 = case shown="0, Default" w2395 {
          tunnel: w2416 -> [_ w2710 _]
          tunnel: w2417 -> [_ _ w2711]
          tunnel: [u32[][] [] ("24-bit pixmap") w2710 w2711] -> w2394
          frame #0 {
          }
          frame #1 {
          }
          frame #2 {
          }
        }
        n1367 = case shown="0, Default" w2391 {
          tunnel: w2416 -> [_ w2707 _]
          tunnel: w2417 -> [_ _ w2708]
          tunnel: [u32[][] [] ("24-bit pixmap") w2707 w2708] -> w2392
          frame #0 {
          }
          frame #1 {
          }
          frame #2 {
          }
        }
        n1368 = case shown="0, Default" w2358 {
          tunnel: w2352 -> [_ w2704 _]
          tunnel: w2351 -> [_ _ w2705]
          tunnel: [u32[][] [] ("24-bit pixmap") w2704 w2705] -> w2359
          frame #0 {
          }
          frame #1 {
          }
          frame #2 {
          }
        }
        n1369 = case shown="2" w2361 {
          tunnel: w2352 -> [_ w2701 _]
          tunnel: w2351 -> [_ _ w2702]
          tunnel: [u32[][] [] ("24-bit pixmap") w2701 w2702] -> w2360
          frame #0 {
          }
          frame #1 {
          }
          frame #2 {
          }
        }
        n1370 = case shown="0, Default" w2373 {
          tunnel: w2352 -> [_ w2698 _]
          tunnel: w2351 -> [_ _ w2699]
          tunnel: [u32[][] [] ("24-bit pixmap") w2698 w2699] -> w2374
          frame #0 {
          }
          frame #1 {
          }
          frame #2 {
          }
        }
        n1371 = case shown="0, Default" w2377 {
          tunnel: w2352 -> [_ w2695 _]
          tunnel: w2351 -> [_ _ w2696]
          tunnel: [u32[][] [] ("24-bit pixmap") w2695 w2696] -> w2376
          frame #0 {
          }
          frame #1 {
          }
          frame #2 {